vi "Dresden R2R Sputter 03.02.2018 IY24.vi"() -> ()   [LabVIEW 2009] (continued)
                          frame #2 {
                            n11736 = local read "Semi"() -> (w18490:bool)
                            n11737 = case shown="False" w18490 {
                              frame #0 {
                                n11738 = while {
                                i -> [w18495]
                                stop <- w18492 stop-if-true
                                n11739 = Greater?(x=w18495, y=90) -> (0:w18493:bool)
                                n11740 = local read "started_up_ch2"() -> (w18491:bool)
                                n11741 = case shown="True" w18493 {
                                frame #0 {
                                }
                                frame #1 {
                                n11742 = local write "Semi"(TRUE ("Semi")) -> ()
                                n11743 = local write "Error Message"("Chamber 2 Pressure is not suitable  \nfor transfer process!\nPlease check connections." ("Error Message")) -> ()
                                }
                                }
                                n11744 = case shown="False" w18491 {
                                tunnel: [FALSE TRUE] -> w18492
                                frame #0 {
                                n11745 = Wait Until Next ms Multiple(millisecond multiple=u32 200) -> ()  [unwired: 1 out]
                                }
                                frame #1 {
                                }
                                }
                                }
                              }
                              frame #1 {
                              }
                            }
                          }
                          frame #3 {
                            n11746 = local read "Semi"() -> (w18501:bool)
                            n11747 = case shown="False" w18501 {
                              frame #0 {
                                n11748 = local write "CH1_2_trns_1"(TRUE ("CH1_2_trns_0")) -> ()
                                n11749 = Wait (ms)(milliseconds to wait=u32 1000) -> ()  [unwired: 1 out]
                              }
                              frame #1 {
                              }
                            }
                          }
                        }
                      }
                      frame #1 {
                      }
                    }
                  }
                  frame #1 {
                  }
                }
              }
              frame #1 {
              }
            }
          }
          frame #4 {
            # "TRNS GV OPEN"
            n11750 = local read "Semi"() -> (w18504:bool)
            n11751 = case shown="False" w18504 {
              frame #0 {
                n11752 = stacked-sequence {
                  frame #0 {
                    n11753 = local read "Semi"() -> (w18505:bool)
                    n11754 = case shown="False" w18505 {
                      frame #0 {
                        n11755 = while {
                          i -> [w18512]
                          stop <- w18507 stop-if-true
                          n11756 = Greater?(x=w18512, y=50) -> (0:w18510:bool)
                          n11757 = local read "Ch1_Trns_gv_bp2_di"() -> (w18506:bool)
                          n11758 = case shown="True" w18510 {
                            frame #0 {
                            }
                            frame #1 {
                              n11759 = local write "Semi"(TRUE ("Semi")) -> ()
                              n11760 = local write "Error Message"("Transfer process was cancelled.\nPlease check CH1-Trns-GV connections." ("Error Message")) -> ()
                            }
                          }
                          n11761 = case shown="False" w18506 {
                            tunnel: [FALSE TRUE] -> w18509
                            frame #0 {
                              n11762 = Wait Until Next ms Multiple(millisecond multiple=u32 200) -> ()  [unwired: 1 out]
                              n11763 = local write "Ch1_Trns_gv_bp2_do"(TRUE ("Ch1_pet_cool_up_do")) -> ()
                            }
                            frame #1 {
                            }
                          }
                          n11764 = local read "Semi"() -> (w18508:bool)
                          n11765 = Or(x=w18509, y=w18508) -> (x .or. y?=w18507:bool)
                        }
                      }
                      frame #1 {
                      }
                    }
                  }
                  frame #1 {
                    n11766 = local read "Semi"() -> (w18519:bool)
                    n11767 = case shown="False" w18519 {
                      frame #0 {
                        n11768 = Wait (ms)(milliseconds to wait=u32 500) -> ()  [unwired: 1 out]
                      }
                      frame #1 {
                      }
                    }
                  }
                  frame #2 {
                    n11769 = local read "Semi"() -> (w18521:bool)
                    n11770 = case shown="False" w18521 {
                      frame #0 {
                        n11771 = while {
                          i -> [w18528]
                          stop <- w18523 stop-if-true
                          n11772 = Greater?(x=w18528, y=50) -> (0:w18526:bool)
                          n11773 = local read "Ch2_trns_gv_bp_di"() -> (w18522:bool)
                          n11774 = case shown="True" w18526 {
                            frame #0 {
                            }
                            frame #1 {
                              n11775 = local write "Semi"(TRUE ("Semi")) -> ()
                              n11776 = local write "Error Message"("Transfer process was cancelled.\nPlease check CH1-Trns-GV connections." ("Error Message")) -> ()
                            }
                          }
                          n11777 = case shown="False" w18522 {
                            tunnel: [FALSE TRUE] -> w18525
                            frame #0 {
                              n11778 = Wait Until Next ms Multiple(millisecond multiple=u32 200) -> ()  [unwired: 1 out]
                              n11779 = local write "Ch2_trns_gv_bp_do"(TRUE ("Ch1_pet_cool_up_do")) -> ()
                            }
                            frame #1 {
                            }
                          }
                          n11780 = local read "Semi"() -> (w18524:bool)
                          n11781 = Or(x=w18525, y=w18524) -> (x .or. y?=w18523:bool)
                        }
                      }
                      frame #1 {
                      }
                    }
                  }
                  frame #3 {
                    n11782 = local read "Semi"() -> (w18535:bool)
                    n11783 = case shown="False" w18535 {
                      frame #0 {
                        n11784 = Wait (ms)(milliseconds to wait=u32 500) -> ()  [unwired: 1 out]
                      }
                      frame #1 {
                      }
                    }
                  }
                }
              }
              frame #1 {
              }
            }
          }
          frame #5 {
            # "TRNS GV OPEN"
            n11785 = local read "Semi"() -> (w18537:bool)
            n11786 = case shown="False" w18537 {
              frame #0 {
                n11787 = stacked-sequence {
                  frame #0 {
                    n11788 = local read "Semi"() -> (w18538:bool)
                    n11789 = case shown="False" w18538 {
                      frame #0 {
                        n11790 = local write "Ch1_Trns_gv_close_do"(FALSE ("Ch1_pet_cool_up_do")) -> ()
                      }
                      frame #1 {
                      }
                    }
                  }
                  frame #1 {
                    n11791 = local read "Semi"() -> (w18540:bool)
                    n11792 = case shown="False" w18540 {
                      frame #0 {
                        n11793 = while {
                          i -> [w18547]
                          stop <- w18542 stop-if-true
                          n11794 = Greater?(x=w18547, y=500) -> (0:w18545:bool)
                          n11795 = local read "Ch1_Trns_gv_open_di"() -> (w18541:bool)
                          n11796 = case shown="True" w18545 {
                            frame #0 {
                            }
                            frame #1 {
                              n11797 = local write "Semi"(TRUE ("Semi")) -> ()
                              n11798 = local write "Error Message"("Transfer process was cancelled.\nPlease check CH1-Trns-GV connections." ("Error Message")) -> ()
                            }
                          }
                          n11799 = case shown="False" w18541 {
                            tunnel: [FALSE TRUE] -> w18544
                            frame #0 {
                              n11800 = Wait Until Next ms Multiple(millisecond multiple=u32 200) -> ()  [unwired: 1 out]
                              n11801 = local write "Ch1_Trns_gv_open_do"(TRUE ("Ch1_pet_cool_up_do")) -> ()
                            }
                            frame #1 {
                            }
                          }
                          n11802 = local read "Semi"() -> (w18543:bool)
                          n11803 = Or(x=w18544, y=w18543) -> (x .or. y?=w18542:bool)
                        }
                      }
                      frame #1 {
                      }
                    }
                  }
                  frame #2 {
                    n11804 = local read "Semi"() -> (w18554:bool)
                    n11805 = case shown="False" w18554 {
                      frame #0 {
                        n11806 = local write "CH1_2trns_2"(TRUE ("CH1_2trns_5")) -> ()
                        n11807 = Wait (ms)(milliseconds to wait=u32 500) -> ()  [unwired: 1 out]
                      }
                      frame #1 {
                      }
                    }
                  }
                }
              }
              frame #1 {
              }
            }
          }
          frame #6 {
            # "TRNS GV control Trnsgv 2_3"
            n11808 = local read "Semi"() -> (w18557:bool)
            n11809 = case shown="False" w18557 {
              frame #0 {
                n11810 = stacked-sequence {
                  frame #0 {
                    n11811 = local read "Semi"() -> (w18558:bool)
                    n11812 = case shown="False" w18558 {
                      frame #0 {
                        n11813 = while {
                          i -> [w18565]
                          stop <- w18560 stop-if-true
                          n11814 = Greater?(x=w18565, y=50) -> (0:w18563:bool)
                          n11815 = local read "Ch1_TGV_control_di"() -> (w18559:bool)
                          n11816 = case shown="True" w18563 {
                            frame #0 {
                            }
                            frame #1 {
                              n11817 = local write "Semi"(TRUE ("Semi")) -> ()
                              n11818 = local write "Error Message"("Transfer process was cancelled.\nPlease check TRNS-GV connections." ("Error Message")) -> ()
                            }
                          }
                          n11819 = case shown="True" w18559 {
                            tunnel: [TRUE FALSE] -> w18562
                            frame #0 {
                            }
                            frame #1 {
                              n11820 = Wait Until Next ms Multiple(millisecond multiple=u32 200) -> ()  [unwired: 1 out]
                              n11821 = local write "Ch1_TGV_control_do"(FALSE ("Ch1_pet_cool_up_do")) -> ()
                            }
                          }
                          n11822 = local read "Semi"() -> (w18561:bool)
                          n11823 = Or(x=w18562, y=w18561) -> (x .or. y?=w18560:bool)
                        }
                      }
                      frame #1 {
                      }
                    }
                  }
                  frame #1 {
                    n11824 = local read "Semi"() -> (w18572:bool)
                    n11825 = case shown="False" w18572 {
                      frame #0 {
                        n11826 = local write "CH1_2trns_3"(TRUE ("CH1_2trns_5")) -> ()
                        n11827 = Wait (ms)(milliseconds to wait=u32 500) -> ()  [unwired: 1 out]
                      }
                      frame #1 {
                      }
                    }
                  }
                }
              }
              frame #1 {
              }
            }
          }
          frame #7 {
            # "TRNS GV control Trnsgv 2_3"
            n11828 = local read "Semi"() -> (w18575:bool)
            n11829 = case shown="False" w18575 {
              frame #0 {
                n11830 = stacked-sequence {
                  frame #0 {
                    n11831 = local read "Semi"() -> (w18576:bool)
                    n11832 = case shown="False" w18576 {
                      frame #0 {
                        n11833 = while {
                          i -> [w18583]
                          stop <- w18578 stop-if-true
                          n11834 = Greater?(x=w18583, y=50) -> (0:w18581:bool)
                          n11835 = local read "Ch2_Trns_interlock_di"() -> (w18577:bool)
                          n11836 = case shown="True" w18581 {
                            frame #0 {
                            }
                            frame #1 {
                              n11837 = local write "Semi"(TRUE ("Semi")) -> ()
                              n11838 = local write "Error Message"("Transfer process was cancelled.\nPlease check TRNS-GV connections." ("Error Message")) -> ()
                            }
                          }
                          n11839 = case shown="False" w18577 {
                            tunnel: [w18585 TRUE] -> w18580
                            frame #0 {
                              n11840 = local read "Ch2_TGV_control_di"() -> (w18584:bool)
                              n11841 = case shown="False" w18584 {
                                tunnel: [FALSE TRUE] -> w18585
                                frame #0 {
                                n11842 = Wait Until Next ms Multiple(millisecond multiple=u32 200) -> ()  [unwired: 1 out]
                                n11843 = local write "Ch2_TGV_control_do"(TRUE ("Ch1_pet_cool_up_do")) -> ()
                                }
                                frame #1 {
                                }
                              }
                            }
                            frame #1 {
                            }
                          }
                          n11844 = local read "Semi"() -> (w18579:bool)
                          n11845 = Or(x=w18580, y=w18579) -> (x .or. y?=w18578:bool)
                        }
                      }
                      frame #1 {
                      }
                    }
                  }
                  frame #1 {
                    n11846 = local read "Semi"() -> (w18593:bool)
                    n11847 = case shown="False" w18593 {
                      frame #0 {
                        n11848 = local write "CH1_2trns_3"(TRUE ("CH1_2trns_5")) -> ()
                        n11849 = Wait (ms)(milliseconds to wait=u32 500) -> ()  [unwired: 1 out]
                      }
                      frame #1 {
                      }
                    }
                  }
                }
              }
              frame #1 {
              }
            }
          }
          frame #8 {
            # "TRNS GV control Trnsgv 3_4"
            n11850 = local read "Semi"() -> (w18596:bool)
            n11851 = case shown="False" w18596 {
              frame #0 {
                n11852 = stacked-sequence {
                  frame #0 {
                    n11853 = local read "Semi"() -> (w18597:bool)
                    n11854 = case shown="False" w18597 {
                      frame #0 {
                        n11855 = while {
                          i -> [w18604]
                          stop <- w18599 stop-if-true
                          n11856 = Greater?(x=w18604, y=50) -> (0:w18602:bool)
                          n11857 = local read "Ch3_Trns_interlock_di"() -> (w18598:bool)
                          n11858 = case shown="True" w18602 {
                            frame #0 {
                            }
                            frame #1 {
                              n11859 = local write "Semi"(TRUE ("Semi")) -> ()
                              n11860 = local write "Error Message"("Transfer process was cancelled.\nPlease check TRNS-GV connections." ("Error Message")) -> ()
                            }
                          }
                          n11861 = case shown="False" w18598 {
                            tunnel: [w18606 TRUE] -> w18601
                            frame #0 {
                              n11862 = local read "Ch3_TGV_control_di"() -> (w18605:bool)
                              n11863 = case shown="False" w18605 {
                                tunnel: [FALSE TRUE] -> w18606
                                frame #0 {
                                n11864 = Wait Until Next ms Multiple(millisecond multiple=u32 200) -> ()  [unwired: 1 out]
                                n11865 = local write "Ch3_TGV_control_do"(TRUE ("Ch1_pet_cool_up_do")) -> ()
                                }
                                frame #1 {
                                }
                              }
                            }
                            frame #1 {
                            }
                          }
                          n11866 = local read "Semi"() -> (w18600:bool)
                          n11867 = Or(x=w18601, y=w18600) -> (x .or. y?=w18599:bool)
                        }
                      }
                      frame #1 {
                      }
                    }
                  }
                  frame #1 {
                    n11868 = local read "Semi"() -> (w18614:bool)
                    n11869 = case shown="False" w18614 {
                      frame #0 {
                        n11870 = local write "CH1_2trns_4"(TRUE ("CH1_2trns_5")) -> ()
                        n11871 = Wait (ms)(milliseconds to wait=u32 500) -> ()  [unwired: 1 out]
                      }
                      frame #1 {
                      }
                    }
                  }
                }
              }
              frame #1 {
              }
            }
          }
          frame #9 {
            # "Right slow deactive"
            n11872 = local read "Semi"() -> (w18617:bool)
            n11873 = case shown="False" w18617 {
              frame #0 {
                n11874 = stacked-sequence {
                  frame #0 {
                    n11875 = local read "Semi"() -> (w18618:bool)
                    n11876 = case shown="False" w18618 {
                      frame #0 {
                        n11877 = while {
                          i -> [w18621]
                          stop <- w18622 stop-if-true
                          n11878 = Greater?(x=w18621, y=50) -> (0:w18619:bool)
                          n11879 = local read "Cnt_Right_slow_di"() -> (w18625:bool)
                          n11880 = case shown="True" w18619 {
                            frame #0 {
                            }
                            frame #1 {
                              n11881 = local write "Semi"(TRUE ("Semi")) -> ()
                              n11882 = local write "Error Message"("Transfer process was\ncancelled.Please check right slow sensor." ("Error Message")) -> ()
                            }
                          }
                          n11883 = case shown="False" w18625 {
                            tunnel: [FALSE ("Ch1_pet_cool_up_do") TRUE ("Ch1_pet_cool_up_do")] -> w18624
                            frame #0 {
                              n11884 = Wait Until Next ms Multiple(millisecond multiple=u32 200) -> ()  [unwired: 1 out]
                              n11885 = local write "Cnt_Right_slow_do"(TRUE ("Ch1_pet_cool_up_do")) -> ()
                            }
                            frame #1 {
                            }
                          }
                          n11886 = local read "Semi"() -> (w18623:bool)
                          n11887 = Or(x=w18624, y=w18623) -> (x .or. y?=w18622:bool)
                        }
                      }
                      frame #1 {
                      }
                    }
                  }
                  frame #1 {
                    n11888 = local read "Semi"() -> (w18632:bool)
                    n11889 = case shown="False" w18632 {
                      frame #0 {
                        n11890 = local write "CH1_2trns_5"(TRUE ("CH1_2trns_7")) -> ()
                        n11891 = Wait (ms)(milliseconds to wait=u32 500) -> ()  [unwired: 1 out]
                      }
                      frame #1 {
                      }
                    }
                  }
                }
              }
              frame #1 {
              }
            }
          }
          frame #10 {
            # "Right limit deactive"
            n11892 = local read "Semi"() -> (w18635:bool)
            n11893 = case shown="False" w18635 {
              frame #0 {
                n11894 = stacked-sequence {
                  frame #0 {
                    n11895 = local read "Semi"() -> (w18636:bool)
                    n11896 = case shown="False" w18636 {
                      frame #0 {
                        n11897 = while {
                          i -> [w18637]
                          stop <- w18641 stop-if-true
                          n11898 = Greater?(x=w18637, y=50) -> (0:w18639:bool)
                          n11899 = local read "Cnt_Right_limit_di"() -> (w18643:bool)
                          n11900 = case shown="True" w18639 {
                            frame #0 {
                            }
                            frame #1 {
                              n11901 = local write "Semi"(TRUE ("Semi")) -> ()
                              n11902 = local write "Error Message"("Transfer process was\ncancelled.Please check right limit sensor." ("Error Message")) -> ()
                            }
                          }
                          n11903 = case shown="False" w18643 {
                            tunnel: [FALSE ("Ch1_pet_cool_up_do") TRUE ("Ch1_pet_cool_up_do")] -> w18642
                            frame #0 {
                              n11904 = Wait Until Next ms Multiple(millisecond multiple=u32 200) -> ()  [unwired: 1 out]
                              n11905 = local write "Cnt_Right_limit_do"(TRUE ("Ch1_pet_cool_up_do")) -> ()
                            }
                            frame #1 {
                            }
                          }
                          n11906 = local read "Semi"() -> (w18640:bool)
                          n11907 = Or(x=w18642, y=w18640) -> (x .or. y?=w18641:bool)
                        }
                      }
                      frame #1 {
                      }
                    }
                  }
                  frame #1 {
                    n11908 = local read "Semi"() -> (w18650:bool)
                    n11909 = case shown="False" w18650 {
                      frame #0 {
                        n11910 = local write "CH1_2trns_6"(TRUE ("CH1_2trns_7")) -> ()
                        n11911 = Wait (ms)(milliseconds to wait=u32 500) -> ()  [unwired: 1 out]
                      }
                      frame #1 {
                      }
                    }
                  }
                }
              }
              frame #1 {
              }
            }
          }
          frame #11 {
            # "Left slow deactive"
            n11912 = local read "Semi"() -> (w18653:bool)
            n11913 = case shown="False" w18653 {
              frame #0 {
                n11914 = stacked-sequence {
                  frame #0 {
                    n11915 = local read "Semi"() -> (w18654:bool)
                    n11916 = case shown="False" w18654 {
                      frame #0 {
                        n11917 = while {
                          i -> [w18655]
                          stop <- w18659 stop-if-true
                          n11918 = Greater?(x=w18655, y=50) -> (0:w18657:bool)
                          n11919 = local read "Cnt_Left_slow_di"() -> (w18661:bool)
                          n11920 = case shown="True" w18657 {
                            frame #0 {
                            }
                            frame #1 {
                              n11921 = local write "Semi"(TRUE ("Semi")) -> ()
                              n11922 = local write "Error Message"("Transfer process was\ncancelled.Please check left slow sensor." ("Error Message")) -> ()
                            }
                          }
                          n11923 = case shown="False" w18661 {
                            tunnel: [FALSE ("Ch1_pet_cool_up_do") TRUE ("Ch1_pet_cool_up_do")] -> w18660
                            frame #0 {
                              n11924 = Wait Until Next ms Multiple(millisecond multiple=u32 200) -> ()  [unwired: 1 out]
                              n11925 = local write "Cnt_Left_slow_do"(TRUE ("Ch1_pet_cool_up_do")) -> ()
                            }
                            frame #1 {
                            }
                          }
                          n11926 = local read "Semi"() -> (w18658:bool)
                          n11927 = Or(x=w18660, y=w18658) -> (x .or. y?=w18659:bool)
                        }
                      }
                      frame #1 {
                      }
                    }
                  }
                  frame #1 {
                    n11928 = local read "Semi"() -> (w18668:bool)
                    n11929 = case shown="False" w18668 {
                      frame #0 {
                        n11930 = local write "CH1_2trns_7"(TRUE ("CH1_2trns_6b")) -> ()
                        n11931 = Wait (ms)(milliseconds to wait=u32 500) -> ()  [unwired: 1 out]
                      }
                      frame #1 {
                      }
                    }
                  }
                }
              }
              frame #1 {
              }
            }
          }
          frame #12 {
            # "Left limit deactive"
            n11932 = local read "Semi"() -> (w18671:bool)
            n11933 = case shown="False" w18671 {
              frame #0 {
                n11934 = stacked-sequence {
                  frame #0 {
                    n11935 = local read "Semi"() -> (w18672:bool)
                    n11936 = case shown="False" w18672 {
                      frame #0 {
                        n11937 = while {
                          i -> [w18673]
                          stop <- w18677 stop-if-true
                          n11938 = Greater?(x=w18673, y=50) -> (0:w18675:bool)
                          n11939 = local read "Cnt_Left_limit_di"() -> (w18679:bool)
                          n11940 = case shown="True" w18675 {
                            frame #0 {
                            }
                            frame #1 {
                              n11941 = local write "Semi"(TRUE ("Semi")) -> ()
                              n11942 = local write "Error Message"("Transfer process was\ncancelled.Please check left limit sensor." ("Error Message")) -> ()
                            }
                          }
                          n11943 = case shown="False" w18679 {
                            tunnel: [FALSE ("Ch1_pet_cool_up_do") TRUE ("Ch1_pet_cool_up_do")] -> w18678
                            frame #0 {
                              n11944 = Wait Until Next ms Multiple(millisecond multiple=u32 200) -> ()  [unwired: 1 out]
                              n11945 = local write "Cnt_Left_limit_do"(TRUE ("Ch1_pet_cool_up_do")) -> ()
                            }
                            frame #1 {
                            }
                          }
                          n11946 = local read "Semi"() -> (w18676:bool)
                          n11947 = Or(x=w18678, y=w18676) -> (x .or. y?=w18677:bool)
                        }
                      }
                      frame #1 {
                      }
                    }
                  }
                  frame #1 {
                    n11948 = local read "Semi"() -> (w18686:bool)
                    n11949 = case shown="False" w18686 {
                      frame #0 {
                        n11950 = local write "CH1_2trns_8"(TRUE ("CH1_2trns_6c")) -> ()
                        n11951 = Wait (ms)(milliseconds to wait=u32 500) -> ()  [unwired: 1 out]
                      }
                      frame #1 {
                      }
                    }
                  }
                }
              }
              frame #1 {
              }
            }
          }
          frame #13 {
            # "Casette Direction"
            n11952 = local read "Semi"() -> (w18689:bool)
            n11953 = case shown="False" w18689 {
              frame #0 {
                n11954 = stacked-sequence {
                  frame #0 {
                    n11955 = local read "Semi"() -> (w18690:bool)
                    n11956 = case shown="False" w18690 {
                      frame #0 {
                        n11957 = while {
                          i -> [w18696]
                          stop <- w18691 stop-if-true
                          n11958 = Greater?(x=w18696, y=50) -> (0:w18697:bool)
                          n11959 = case shown="True" w18697 {
                            frame #0 {
                            }
                            frame #1 {
                              n11960 = local write "Semi"(TRUE ("Semi")) -> ()
                              n11961 = local write "Error Message"("Transfer process was cancelled.\nPlease check Casette Direction connections." ("Error Message")) -> ()
                            }
                          }
                          n11962 = local read "Casette_servo_left_direction_di"() -> (w18694:bool)
                          n11963 = case shown="True" w18694 {
                            tunnel: [TRUE ("Casette_servo_left_direction_do") FALSE ("Casette_servo_left_direction_do")] -> w18693
                            frame #0 {
                            }
                            frame #1 {
                              n11964 = Wait Until Next ms Multiple(millisecond multiple=u32 200) -> ()  [unwired: 1 out]
                              n11965 = local write "Casette_servo_left_direction_do"(FALSE ("Casette_servo_left_direction_do")) -> ()
                            }
                          }
                          n11966 = local read "Semi"() -> (w18692:bool)
                          n11967 = Or(x=w18693, y=w18692) -> (x .or. y?=w18691:bool)
                        }
                      }
                      frame #1 {
                      }
                    }
                  }
                  frame #1 {
                    n11968 = local read "Semi"() -> (w18704:bool)
                    n11969 = case shown="False" w18704 {
                      frame #0 {
                        n11970 = local write "CH1_2trns_9"(TRUE ("CH1_2trns_7")) -> ()
                        n11971 = Wait (ms)(milliseconds to wait=u32 500) -> ()  [unwired: 1 out]
                      }
                      frame #1 {
                      }
                    }
                  }
                }
              }
              frame #1 {
              }
            }
          }
          frame #14 {
            # "SET CASSETTE SERVO  SPEED 300"
            n11972 = local read "Semi"() -> (w18707:bool)
            n11973 = case shown="False" w18707 {
              frame #0 {
                n11974 = stacked-sequence {
                  frame #0 {
                    n11975 = local read "Semi"() -> (w18708:bool)
                    n11976 = case shown="False" w18708 {
                      frame #0 {
                        n11977 = local write "Cassette_servo_speed_value"(u16 300 ("Cassette_servo_speed_value")) -> ()
                      }
                      frame #1 {
                      }
                    }
                  }
                  frame #1 {
                    n11978 = local read "Semi"() -> (w18710:bool)
                    n11979 = case shown="False" w18710 {
                      frame #0 {
                        n11980 = Wait (ms)(milliseconds to wait=u32 200) -> ()  [unwired: 1 out]
                      }
                      frame #1 {
                      }
                    }
                  }
                  frame #2 {
                    n11981 = local read "Semi"() -> (w18712:bool)
                    n11982 = case shown="False" w18712 {
                      frame #0 {
                        n11983 = local write "Cassette_servo_speed_auto_set"(TRUE ("Cassette_servo_speed_set")) -> ()
                      }
                      frame #1 {
                      }
                    }
                  }
                  frame #3 {
                    n11984 = local read "Semi"() -> (w18714:bool)
                    n11985 = case shown="False" w18714 {
                      frame #0 {
                        n11986 = Wait (ms)(milliseconds to wait=u32 200) -> ()  [unwired: 1 out]
                      }
                      frame #1 {
                      }
                    }
                  }
                  frame #4 {
                    n11987 = local read "Semi"() -> (w18716:bool)
                    n11988 = case shown="False" w18716 {
                      frame #0 {
                        n11989 = local write "CH1_2trns_10"(TRUE ("CH1_2trns_7")) -> ()
                        n11990 = Wait (ms)(milliseconds to wait=u32 500) -> ()  [unwired: 1 out]
                      }
                      frame #1 {
                      }
                    }
                  }
                }
              }
              frame #1 {
              }
            }
          }
          frame #15 {
            # "Casette Servo Start"
            n11991 = local read "Semi"() -> (w18719:bool)
            n11992 = case shown="False" w18719 {
              frame #0 {
                n11993 = stacked-sequence {
                  frame #0 {
                    n11994 = while {
                      i -> [w18725]
                      stop <- w18720 stop-if-true
                      n11995 = Greater?(x=w18725, y=50) -> (0:w18726:bool)
                      n11996 = local read "Casette_servo_start/stop_di"() -> (w18723:bool)
                      n11997 = case shown="True" w18726 {
                        frame #0 {
                        }
                        frame #1 {
                          n11998 = local write "Semi"(TRUE ("Semi")) -> ()
                          n11999 = local write "Error Message"("Transfer process was cancelled.\nPlease check Casette connections." ("Error Message")) -> ()
                        }
                      }
                      n12000 = case shown="False" w18723 {
                        tunnel: [FALSE ("Casette_servo_left_direction_do") TRUE ("Casette_servo_left_direction_do")] -> w18722
                        frame #0 {
                          n12001 = Wait Until Next ms Multiple(millisecond multiple=u32 200) -> ()  [unwired: 1 out]
                          n12002 = local write "Casette_servo_start/stop_do"(TRUE ("Casette_servo_left_direction_do")) -> ()
                        }
                        frame #1 {
                        }
                      }
                      n12003 = local read "Semi"() -> (w18721:bool)
                      n12004 = Or(x=w18722, y=w18721) -> (x .or. y?=w18720:bool)
                    }
                  }
                  frame #1 {
                    n12005 = local read "Semi"() -> (w18733:bool)
                    n12006 = case shown="False" w18733 {
                      frame #0 {
                        n12007 = local write "CH1_2trns_11"(TRUE ("CH1_2trns_9")) -> ()
                        n12008 = Wait (ms)(milliseconds to wait=u32 500) -> ()  [unwired: 1 out]
                      }
                      frame #1 {
                      }
                    }
                  }
                }
              }
              frame #1 {
              }
            }
          }
          frame #16 {
            # "Right sensors activate"
            n12009 = local read "Semi"() -> (w18736:bool)
            n12010 = case shown="False" w18736 {
              frame #0 {
                n12011 = stacked-sequence {
                  frame #0 {
                    n12012 = while {
                      i -> [w18745]
                      stop <- w18741 stop-if-true
                      n12013 = local read "Counter_read_data"() -> (w18738:i16)
                      n12014 = Greater?(x=w18745, y=1500) -> (0:w18744:bool)
                      n12015 = case shown="True" w18744 {
                        frame #0 {
                        }
                        frame #1 {
                          n12016 = local write "Semi"(TRUE ("Semi")) -> ()
                          n12017 = local write "Error Message"("Transfer process was cancelled.\nPlease check Casette & Sensor\nconnections." ("Error Message")) -> ()
                        }
                      }
                      n12018 = Less Or Equal?(x=w18738, y=i16 800) -> (x <= y?=w18739:bool)
                      n12019 = case shown="False" w18739 {
                        tunnel: [FALSE TRUE] -> w18742
                        frame #0 {
                          n12020 = Wait Until Next ms Multiple(millisecond multiple=u32 200) -> ()  [unwired: 1 out]
                        }
                        frame #1 {
                        }
                      }
                      n12021 = local read "Semi"() -> (w18740:bool)
                      n12022 = Or(x=w18742, y=w18740) -> (x .or. y?=w18741:bool)
                    }
                  }
                  frame #1 {
                    n12023 = while {
                      i -> [w18754]
                      stop <- w18751 stop-if-true
                      n12024 = Greater?(x=w18754, y=50) -> (0:w18755:bool)
                      n12025 = local read "Cnt_Right_slow_di"() -> (w18757:bool)
                      n12026 = case shown="True" w18755 {
                        frame #0 {
                        }
                        frame #1 {
                          n12027 = local write "Semi"(TRUE ("Semi")) -> ()
                          n12028 = local write "Error Message"("\nPlease check connections." ("Error Message")) -> ()
                        }
                      }
                      n12029 = case shown="True" w18757 {
                        tunnel: [TRUE ("Cnt_Left_slow_do") FALSE ("Cnt_Left_slow_do")] -> w18753
                        frame #0 {
                        }
                        frame #1 {
                          n12030 = local write "Cnt_Right_slow_do"(FALSE ("Cnt_Left_slow_do")) -> ()
                          n12031 = Wait Until Next ms Multiple(millisecond multiple=u32 200) -> ()  [unwired: 1 out]
                        }
                      }
                      n12032 = local read "Semi"() -> (w18752:bool)
                      n12033 = Or(x=w18753, y=w18752) -> (x .or. y?=w18751:bool)
                    }
                  }
                  frame #2 {
                    n12034 = while {
                      i -> [w18767]
                      stop <- w18764 stop-if-true
                      n12035 = Greater?(x=w18767, y=50) -> (0:w18768:bool)
                      n12036 = local read "Cnt_Right_limit_di"() -> (w18770:bool)
                      n12037 = case shown="True" w18768 {
                        frame #0 {
                        }
                        frame #1 {
                          n12038 = local write "Semi"(TRUE ("Semi")) -> ()
                          n12039 = local write "Error Message"("\nPlease check connections." ("Error Message")) -> ()
                        }
                      }
                      n12040 = case shown="True" w18770 {
                        tunnel: [TRUE ("Cnt_Left_slow_do") FALSE ("Cnt_Left_slow_do")] -> w18766
                        frame #0 {
                        }
                        frame #1 {
                          n12041 = local write "Cnt_Right_limit_do"(FALSE ("Cnt_Left_slow_do")) -> ()
                          n12042 = Wait Until Next ms Multiple(millisecond multiple=u32 200) -> ()  [unwired: 1 out]
                        }
                      }
                      n12043 = local read "Semi"() -> (w18765:bool)
                      n12044 = Or(x=w18766, y=w18765) -> (x .or. y?=w18764:bool)
                    }
                  }
                  frame #3 {
                    n12045 = local read "Semi"() -> (w18777:bool)
                    n12046 = case shown="False" w18777 {
                      frame #0 {
                        n12047 = local write "CH1_2trns_12"(TRUE ("CH1_2trns_11")) -> ()
                        n12048 = Wait (ms)(milliseconds to wait=u32 500) -> ()  [unwired: 1 out]
                      }
                      frame #1 {
                      }
                    }
                  }
                }
              }
              frame #1 {
              }
            }
          }
          frame #17 {
            # "SET CASSETTE SERVO  SPEED 100"
            n12049 = local read "Semi"() -> (w18780:bool)
            n12050 = case shown="False" w18780 {
              frame #0 {
                n12051 = stacked-sequence {
                  frame #0 {
                    n12052 = while {
                      i -> [w18787]
                      stop <- w18783 stop-if-true
                      n12053 = local read "Ch1_Right_slow_di"() -> (w18781:bool)
                      n12054 = Greater?(x=w18787, y=1500) -> (0:w18786:bool)
                      n12055 = case shown="True" w18786 {
                        frame #0 {
                        }
                        frame #1 {
                          n12056 = local write "Semi"(TRUE ("Semi")) -> ()
                          n12057 = local write "Error Message"("Transfer process was cancelled.\nPlease check Casette & Sensor\nconnections." ("Error Message")) -> ()
                        }
                      }
                      n12058 = case shown="False" w18781 {
                        tunnel: [FALSE TRUE] -> w18784
                        frame #0 {
                          n12059 = Wait Until Next ms Multiple(millisecond multiple=u32 200) -> ()  [unwired: 1 out]
                        }
                        frame #1 {
                        }
                      }
                      n12060 = local read "Semi"() -> (w18782:bool)
                      n12061 = Or(x=w18784, y=w18782) -> (x .or. y?=w18783:bool)
                    }
                  }
                  frame #1 {
                    n12062 = disable-structure shown="Disabled" {
                      frame #0 {
                        n12063 = while {
                          i -> [w18802]
                          stop <- w18798 stop-if-true
                          n12064 = local read "Counter_read_data"() -> (w18795:i16)
                          n12065 = Greater?(x=w18802, y=5000) -> (0:w18801:bool)
                          n12066 = case shown="True" w18801 {
                            frame #0 {
                            }
                            frame #1 {
                              n12067 = local write "Semi"(TRUE ("Semi")) -> ()
                            }
                          }
                          n12068 = In Range and Coerce(upper limit=i16 1990, x=w18795, lower limit=i16 1980 ("upper limit")) -> (In Range?=w18793:bool)  [unwired: 1 out]
                          n12069 = case shown="True" w18793 {
                            tunnel: [FALSE TRUE] -> w18799
                            frame #0 {
                              n12070 = Wait Until Next ms Multiple(millisecond multiple=u32 200) -> ()  [unwired: 1 out]
                            }
                            frame #1 {
                            }
                          }
                          n12071 = local read "Semi"() -> (w18797:bool)